vi "UHR-Fleezers Control (host) - 12.4.vi"() -> ()   [LabVIEW 2012] (continued)
        n1557 = Divide(x=w2246, y=w2245) -> (x/y=w2244:dbl)
        n1558 = Multiply(x=i16 10, y=w2223) -> (x*y=w2221:i16)
        n1559 = Multiply(x="N APD Samp/step", y=w2244) -> (x*y=w2243:dbl)
        "Cycles/step (MCL)" <- w2243
        n1560 = Divide(x=w2221, y=w2220) -> (x/y=→"Actual MCL Inc (V)":dbl)
        n1561 = Multiply(x="N APD Samp/step", y="Scan steps (MCL)") -> (x*y=w2235:dbl)
        n1562 = local read "APD Samples/FIFO Acq."() -> (w2232:dbl)
        n1563 = Multiply(x=w2235, y=u64 2) -> (x*y=w2234:dbl)
        "Data points/scan (f+b)" <- w2234
        n1564 = Multiply(x=w2234, y=w2225) -> (x*y=w2252:dbl)
        "Data points/scans (MCL)" <- w2252
        n1565 = Multiply(x=w2233, y=w2234) -> (x*y=w2226:dbl)
        "Time/f+b scan (s) (MCL)" <- w2226
        n1566 = Divide(x=w2252, y=w2232) -> (x/y=→"N sets should be saved (MCL)":dbl)
        n1567 = Multiply(x=w2226, y=w2225) -> (x*y=→"Total Time (s)":dbl)
        n1568 = Not(x="Fast Scan Dir") -> (.not. x?=w2230:bool)
        n1569 = xnode "Read/Write Control"("FPGA VI Reference In"=w2256, "error in"=w2255, "Scan steps (MCL)"="Scan steps (MCL)", "Number of scans (MCL)"=w2225, "Cycles per step (MCL)"=w2243, "Scan freq.  increment (MCL)"=w2223, "1D or 2D Scan?"="2D or 1D Scan", "MCL Scan Axis"=w2230, "Cont. Scan (MCL)"="Continuous MCL Scanning") -> ("error out"=w2254:errorcluster)  [unwired: 1 out]
      }
      event "Read Cal": Value Change {
        w2258 = 1000.0 ("y")
        n1570 = event-data() -> ()  [unwired: 7 out]
        n1571 = local read "Save file name"() -> (w2283:path)
        n1572 = local write "Read Cal"(FALSE ("Read Cal")) -> ()
        n1573 = Strip Path(path=w2283) -> (stripped path=w2282:path)  [unwired: 1 out]
        n1574 = Path To String(path=w2282) -> (string=w2281:string)
        n1575 = Concatenate Strings(w2281, "\\current.cal" ("string")) -> (w2279:string)
        n1576 = String To Path(string=w2279) -> (path=w2278:path)
        n1577 = Open/Create/Replace File(file path (use dialog)=w2278, operation (0:open)=T27."open", access (0:read/write)=enum16{"read/write", "read-only", "write-only"}."read-only") -> (refnum out=w2286:refnum<file>, error out=w2272:errorcluster)  [unwired: 1 in, 3 out]
        n1578 = Deny Access(4:w2272, 7:w2286) -> (0:w2271:errorcluster, 3:w2277:refnum<file>)  [unwired: 1 out]
        n1579 = Read from Binary File(5:0.0, 8:w2271, 9:T26."big-endian, network order" ("byte order (0:big-endian, network order)"), 10:-1 ("count (1)"), 11:w2277) -> (0:w2270:errorcluster, 2:w2268:dbl[], 3:w2273:refnum<file>)  [unwired: 2 out]
        n1580 = Array To Cluster(array=w2268) -> (cluster=w2267:T29)
        n1581 = Unbundle(w2267) -> ("[0]"=w2266:dbl, "[1]"=w2265:dbl, "[2]"=w2264:dbl, "[3]"=w2263:dbl, "[4]"=w2262:dbl, "[5]"=w2261:dbl)
        n1582 = Close File(refnum=w2273, error in=w2270) -> (error out=→"Read cal error":errorcluster)  [unwired: 1 out]
        n1583 = Multiply(x=w2261, y=w2258) -> (x*y=w2259:dbl)
        n1584 = local write "T2 kappa_x (pN/nm)"(w2263) -> ()
        n1585 = local write "T1 kappa_x (pN/nm)"(w2264) -> ()
        n1586 = local write "T1 alpha_x (nm/V)"(w2266) -> ()
        n1587 = local write "T2 alpha_x (nm/V)"(w2265) -> ()
        n1588 = Multiply(x=w2262, y=w2258) -> (x*y=w2260:dbl)
        n1589 = local write "T1 offset_x (mV)"(w2260) -> ()
        n1590 = local write "T2 offset_x (mV)"(w2259) -> ()
      }
      event "Abort MCL Scan": Value Change {
        n1591 = event-data() -> ()  [unwired: 7 out]
        n1592 = local write "MCL Scanning"(FALSE ("MCL Scanning")) -> ()
        n1593 = xnode "Read/Write Control"("FPGA VI Reference In"=w2291, "error in"=w2290, "Abort scan (MCL)"="Abort MCL Scan") -> ("error out"=w2289:errorcluster)  [unwired: 1 out]
      }
      event "Update Count (MCL)": Value Change {
        n1594 = event-data() -> ()  [unwired: 7 out]
        n1595 = xnode "Read/Write Control"("FPGA VI Reference In"=w2295, "error in"=w2294, "MCL count"="Update Count (MCL)") -> ("error out"=w2293:errorcluster)  [unwired: 1 out]
      }
      event "+ phase (MCL)", "- phase (MCL)": Value Change {
        n1596 = event-data() -> ()  [unwired: 7 out]
        n1597 = Or(x="- phase (MCL)", y="+ phase (MCL)") -> (x .or. y?=w2298:bool)
        n1598 = Negate(x="Phase adjust (MCL)") -> (-x=w2304:i16)
        n1599 = Select(t=w2304, s="+ phase (MCL)", f="Phase adjust (MCL)") -> (s? t:f=w2302:i16)
        n1600 = xnode "Read/Write Control"("FPGA VI Reference In"=w2306, "error in"=w2305, "Phase count adjustment (MCL)"=w2302) -> ("FPGA VI Reference Out"=w2299:T19, "error out"=w2300:errorcluster)
        n1601 = xnode "Read/Write Control"("FPGA VI Reference In"=w2299, "error in"=w2300, "+ phase (MCL)"=w2298) -> ("error out"=w2297:errorcluster)  [unwired: 1 out]
      }
      event "Abort AOD Scan": Value Change {
        n1602 = event-data() -> ()  [unwired: 7 out]
        n1603 = xnode "Read/Write Control"("FPGA VI Reference In"=w2310, "error in"=w2309, "Abort scan"="Abort AOD Scan") -> ("error out"=w2308:errorcluster)  [unwired: 1 out]
      }
      event "Continuous AOD Scanning": Value Change {
        n1604 = event-data() -> ()  [unwired: 7 out]
        n1605 = xnode "Read/Write Control"("FPGA VI Reference In"=w2314, "error in"=w2313, "Cont. Scan"="Continuous AOD Scanning") -> ("error out"=w2312:errorcluster)  [unwired: 1 out]
      }
      event "Index": Value Change {
        n1606 = event-data() -> ()  [unwired: 7 out]
        n1607 = call "Create new save file.vi"("Insert"="", "Ext"=".dat" ("string"), "Index In"="Index") -> ("Path Out"=→"Save file name":path, "Index Out"=w2315:dbl)
        "Save index" <- w2315
        n1608 = local write "Index"(w2315) -> ()
      }
      event "AO1", "AO2": Value Change {
        w2330 = 10.0 ("y")
        w2329 = 32767.0 ("y")
        n1609 = event-data() -> ()  [unwired: 7 out]
        n1610 = local read "AO2"() -> (w2328:dbl)
        n1611 = local read "AO1"() -> (w2325:dbl)
        n1612 = Multiply(x=w2325, y=w2329) -> (x*y=w2324:dbl)
        n1613 = Multiply(x=w2328, y=w2329) -> (x*y=w2327:dbl)
        n1614 = Divide(x=w2324, y=w2330) -> (x/y=w2323:dbl)
        n1615 = Divide(x=w2327, y=w2330) -> (x/y=w2326:dbl)
        n1616 = To Word Integer(number=w2323) -> (16bit integer=w2331:i16)
        n1617 = To Word Integer(number=w2326) -> (16bit integer=w2332:i16)
        n1618 = xnode "Read/Write Control"("FPGA VI Reference In"=w2322, "error in"=w2321, "AO1"=w2331, "AO2"=w2332) -> ("error out"=w2320:errorcluster)  [unwired: 1 out]
      }
      event "Inject Pump 1": Value Change {
        n1619 = event-data() -> ()  [unwired: 7 out]
        n1620 = local read "Use Harvard pumps\nfor beads (else Chemyx)"() -> (w2334:bool)
        n1621 = case shown="True" w2334 {
          tunnel: "Inject Pump 1" -> [w2338 w2376]
          tunnel: w2333 -> [_ w2377]
          frame False {
            n1622 = local read "Pump write delay (ms)"() -> (w2337:dbl)
            n1623 = local read "Chemyx Syringe Pump Serial Port"() -> (w2336:refnum<visa-resource-name>)
            n1624 = case shown="True" w2338 {
              tunnel: w2337 -> [w2344 w2358]
              tunnel: w2336 -> [w2341 w2357]
              frame False {
                n1625 = flat-sequence {
                  tunnel: w2341 -> [w2345]
                  tunnel: [w2345] -> w2342
                  tunnel: w2344 -> [_]
                  tunnel: [w2348] -> w2343
                  tunnel: w2342 -> [w2348]
                  tunnel: w2343 -> [w2349]
                  tunnel: [w2349] -> w2339
                  tunnel: [w2351] -> w2340
                  tunnel: w2339 -> [w2351]
                  tunnel: w2340 -> [w2353]
                  frame #0 {
                    n1626 = call "Write to pump.vi"("string"="enter pump1", "VISA resource name"=w2345) -> ()  [unwired: 1 out]
                  }
                  frame #1 {
                    n1627 = Wait (ms)(milliseconds to wait="Pump pause delay (ms)") -> ()  [unwired: 1 out]
                  }
                  frame #2 {
                    n1628 = call "Write to pump.vi"("string"="stop", "VISA resource name"=w2349) -> ()  [unwired: 1 out]
                  }
                  frame #3 {
                    n1629 = Wait (ms)(milliseconds to wait=u32 500) -> ()  [unwired: 1 out]
                  }
                  frame #4 {
                    n1630 = call "Write to pump.vi"("string"="stop", "VISA resource name"=w2353) -> ()  [unwired: 1 out]
                  }
                }
              }
              frame True {
                n1631 = flat-sequence {
                  tunnel: w2357 -> [w2367]
                  tunnel: w2358 -> [w2362]
                  tunnel: w2358 -> [w2369]
                  tunnel: w2357 -> [w2370]
                  tunnel: [w2370] -> w2355
                  tunnel: [w2372] -> w2356
                  tunnel: w2355 -> [w2372]
                  tunnel: w2356 -> [w2374]
                  frame #0 {
                    n1632 = local read "All Pump Parameters"() -> (w2361:T5)
                    n1633 = Unbundle By Name(w2361) -> ("Pump 1"=w2368:T30)
                    n1634 = call "Set pump parameters.vi"("Pump write delay (ms)"=w2362, "Volume (uL)"="Ch 1 Inject Volume (uL)", "Rate (uL/h)"="Ch 1 Inject Rate (ul/h)", "Units"=4.0, "Pump #"=1.0, "Pump Parameters In"=w2368, "VISA resource name"=w2367) -> ("Pump Parameters Out"=w2360:T30)  [unwired: 3 in]
                    n1635 = Bundle By Name(cluster=w2361, "Pump 1"=w2360) -> (w2359:T5)
                    n1636 = local write "All Pump Parameters"(w2359) -> ()
                  }
                  frame #1 {
                    n1637 = Wait (ms)(milliseconds to wait=w2369) -> ()  [unwired: 1 out]
                  }
                  frame #2 {
                    n1638 = call "Write to pump.vi"("string"="start", "VISA resource name"=w2370) -> ()  [unwired: 1 out]
                  }
                  frame #3 {
                    n1639 = Wait (ms)(milliseconds to wait=u32 500) -> ()  [unwired: 1 out]
                  }
                  frame #4 {
                    n1640 = call "Write to pump.vi"("string"="start", "VISA resource name"=w2374) -> ()  [unwired: 1 out]
                  }
                }
              }
            }
          }
          frame True {
            n1641 = case shown="False" w2376 {
              tunnel: w2377 -> [w2378 w2388]
              frame False {
                n1642 = flat-sequence {
                  tunnel: w2378 -> [w2380]
                  frame #0 {
                    n1643 = local write "Flushing P1"(FALSE ("Flushing P1")) -> ()
                    n1644 = Concatenate Strings("stop" ("string"), "\r") -> (w2382:string)
                    n1645 = VISA Write(VISA resource name=w2380, write buffer=w2382) -> ()  [unwired: 1 in, 3 out]
                  }
                  frame #1 {
                    n1646 = property on="Clear Volume P1" class="Bool (strict)"("Val(Sgnl)"=TRUE ("Value (Signaling)")) -> ()  [unwired: 2 in, 2 out]
                  }
                }
              }
              frame True {
                n1647 = local read "Normal Flow Rate (ul/h) P1"() -> (w2386:dbl)
                n1648 = Number To Decimal String(number=w2386) -> (decimal integer string=w2392:string)  [unwired: 1 in]
                n1649 = Concatenate Strings("irate  " ("string"), w2392, " u/h" ("string"), "\r") -> (w2390:string)
                n1650 = VISA Write(VISA resource name=w2388, write buffer=w2390) -> (VISA resource name out=w2387:refnum<visa-resource-name>)  [unwired: 1 in, 2 out]
                n1651 = Concatenate Strings("irun" ("string"), "\r") -> (w2394:string)
                n1652 = VISA Write(VISA resource name=w2387, write buffer=w2394) -> ()  [unwired: 1 in, 3 out]
              }
            }
          }
        }
      }
      event "Inject Pump 3": Value Change {
        n1653 = event-data() -> ()  [unwired: 7 out]
        n1654 = local read "Use Harvard pumps\nfor beads (else Chemyx)"() -> (w2397:bool)
        n1655 = case shown="True" w2397 {
          tunnel: "Inject Pump 3" -> [w2401 w2440]
          tunnel: w2396 -> [_ w2439]
          frame False {
            n1656 = local read "Pump write delay (ms)"() -> (w2400:dbl)
            n1657 = case shown="True" w2401 {
              tunnel: w2400 -> [w2407 w2421]
              tunnel: "Chemyx Syringe Pump Serial Port" -> [w2404 w2420]
              frame False {
                n1658 = flat-sequence {
                  tunnel: w2404 -> [w2408]
                  tunnel: [w2408] -> w2405
                  tunnel: w2407 -> [_]
                  tunnel: [w2411] -> w2406
                  tunnel: w2405 -> [w2411]
                  tunnel: w2406 -> [w2412]
                  tunnel: [w2412] -> w2402
                  tunnel: [w2414] -> w2403
                  tunnel: w2402 -> [w2414]
                  tunnel: w2403 -> [w2416]
                  frame #0 {
                    n1659 = call "Write to pump.vi"("string"="enter pump3", "VISA resource name"=w2408) -> ()  [unwired: 1 out]
                  }
                  frame #1 {
                    n1660 = local read "Pump pause delay (ms)"() -> (w2410:u32)
                    n1661 = Wait (ms)(milliseconds to wait=w2410) -> ()  [unwired: 1 out]
                  }
                  frame #2 {
                    n1662 = call "Write to pump.vi"("string"="stop", "VISA resource name"=w2412) -> ()  [unwired: 1 out]
                  }
                  frame #3 {
                    n1663 = Wait (ms)(milliseconds to wait=u32 0) -> ()  [unwired: 1 out]
                  }
                  frame #4 {
                    n1664 = call "Write to pump.vi"("string"="stop", "VISA resource name"=w2416) -> ()  [unwired: 1 out]
                  }
                }
              }
              frame True {
                n1665 = flat-sequence {
                  tunnel: w2420 -> [w2430]
                  tunnel: w2421 -> [w2425]
                  tunnel: w2421 -> [w2432]
                  tunnel: w2420 -> [w2433]
                  tunnel: [w2433] -> w2419
                  tunnel: [w2436] -> w2418
                  tunnel: w2419 -> [w2436]
                  tunnel: w2418 -> [w2437]
                  frame #0 {
                    n1666 = local read "All Pump Parameters"() -> (w2424:T5)
                    n1667 = Unbundle By Name(w2424) -> ("Pump 3"=w2431:T30)
                    n1668 = call "Set pump parameters.vi"("Pump write delay (ms)"=w2425, "Volume (uL)"="Ch 3 Inject Volume (uL)", "Rate (uL/h)"="Ch 3 Inject Rate (ul/h)", "Units"=4.0, "Pump #"=3.0, "Pump Parameters In"=w2431, "VISA resource name"=w2430) -> ("Pump Parameters Out"=w2423:T30)  [unwired: 3 in]
                    n1669 = Bundle By Name(cluster=w2424, "Pump 3"=w2423) -> (w2422:T5)
                    n1670 = local write "All Pump Parameters"(w2422) -> ()
                  }
                  frame #1 {
                    n1671 = Wait (ms)(milliseconds to wait=w2432) -> ()  [unwired: 1 out]
                  }
                  frame #2 {
                    n1672 = call "Write to pump.vi"("string"="start", "VISA resource name"=w2433) -> ()  [unwired: 1 out]
                  }
                  frame #3 {
                    n1673 = Wait (ms)(milliseconds to wait=u32 500) -> ()  [unwired: 1 out]
                  }
                  frame #4 {
                    n1674 = call "Write to pump.vi"("string"="start", "VISA resource name"=w2437) -> ()  [unwired: 1 out]
                  }
                }
              }
            }
          }
          frame True {
            n1675 = case shown="False" w2440 {
              tunnel: w2439 -> [w2441 w2448]
              frame False {
                n1676 = flat-sequence {
                  tunnel: w2441 -> [w2443]
                  frame #0 {
                    n1677 = local write "Flushing P3"(FALSE ("Flushing P3")) -> ()
                    n1678 = Concatenate Strings("stop" ("string"), "\r") -> (w2445:string)
                    n1679 = VISA Write(VISA resource name=w2443, write buffer=w2445) -> ()  [unwired: 1 in, 3 out]
                  }
                  frame #1 {
                    n1680 = property on="Clear Volume P3" class="Bool (strict)"("Val(Sgnl)"=TRUE ("Value (Signaling)")) -> ()  [unwired: 2 in, 2 out]
                  }
                }
              }
              frame True {
                n1681 = local read "Normal Flow Rate (ul/h) P3"() -> (w2449:dbl)
                n1682 = Number To Decimal String(number=w2449) -> (decimal integer string=w2455:string)  [unwired: 1 in]
                n1683 = Concatenate Strings("irate  " ("string"), w2455, " u/h" ("string"), "\r") -> (w2453:string)
                n1684 = VISA Write(VISA resource name=w2448, write buffer=w2453) -> (VISA resource name out=w2451:refnum<visa-resource-name>)  [unwired: 1 in, 2 out]
                n1685 = Concatenate Strings("irun" ("string"), "\r") -> (w2457:string)
                n1686 = VISA Write(VISA resource name=w2451, write buffer=w2457) -> ()  [unwired: 1 in, 3 out]
              }
            }
          }
        }
      }
      event "Inject Pump 2": Value Change {
        n1687 = event-data() -> ()  [unwired: 7 out]
        n1688 = local read "Pump write delay (ms)"() -> (w2461:dbl)
        n1689 = flat-sequence {
          tunnel: w2459 -> [w2474]
          tunnel: w2461 -> [w2470]
          tunnel: "Inject Pump 2" -> [_]
          tunnel: w2461 -> [w2476]
          tunnel: w2459 -> [w2477]
          frame #0 {
            n1690 = local read "All Pump Parameters"() -> (w2469:T5)
            n1691 = Multiply(x=60.0, y="Flush Center Ch Rate (ul/m)") -> (x*y=w2466:dbl)
            n1692 = Unbundle By Name(w2469) -> ("Pump 2"=w2475:T30)
            n1693 = call "Set pump parameters.vi"("Pump write delay (ms)"=w2470, "Volume (uL)"="Flush Center Ch Volume (uL)", "Rate (uL/h)"=w2466, "Units"=3.0, "Pump #"=2.0, "Pump Parameters In"=w2475, "VISA resource name"=w2474) -> ("Pump Parameters Out"=w2468:T30)  [unwired: 3 in]
            n1694 = Bundle By Name(cluster=w2469, "Pump 2"=w2468) -> (w2467:T5)
            n1695 = local write "All Pump Parameters"(w2467) -> ()
            n1696 = Add(x="Flush Center Ch Volume (uL)", y="Total Volume\nFlushed (uL)") -> (x+y=w2463:dbl)
            n1697 = local write "Total Volume\nFlushed (uL)"(w2463) -> ()
          }
          frame #1 {
            n1698 = Wait (ms)(milliseconds to wait=w2476) -> ()  [unwired: 1 out]
          }
          frame #2 {
            n1699 = call "Write to pump.vi"("string"="start", "VISA resource name"=w2477) -> ()  [unwired: 1 out]
          }
        }
        n1700 = local read "Chemyx Syringe Pump Serial Port"() -> (w2459:refnum<visa-resource-name>)
      }
      event "Sample Channel\nFlow": Value Change {
        n1701 = event-data() -> ()  [unwired: 7 out]
        n1702 = Select(t="irun" ("string"), s="Sample Channel\nFlow", f="stop" ("string")) -> (s? t:f=w2481:string)
        n1703 = Concatenate Strings(w2481, "\r") -> (w2484:string)
        n1704 = VISA Write(VISA resource name=w2479, write buffer=w2484) -> ()  [unwired: 1 in, 3 out]
      }
      event "Start Flow": Value Change {
        n1705 = event-data() -> ()  [unwired: 7 out]
        n1706 = local write "Sample Channel\nFlow"(TRUE ("Sample Channel\nFlow")) -> ()
        n1707 = local write "Start Flow"(FALSE ("Start Flow")) -> ()
        n1708 = Concatenate Strings("irun" ("string"), "\r") -> (w2490:string)
        n1709 = VISA Write(VISA resource name=w2486, write buffer=w2490) -> ()  [unwired: 1 in, 3 out]
      }
      event "Stop Flow": Value Change {
        w2492 = FALSE ("Stop Flow")
        n1710 = event-data() -> ()  [unwired: 7 out]
        n1711 = local write "Stop Flow"(w2492) -> ()
        n1712 = local write "Sample Channel\nFlow"(w2492) -> ()
        n1713 = Concatenate Strings("stop" ("string"), "\r") -> (w2495:string)
        n1714 = VISA Write(VISA resource name=w2493, write buffer=w2495) -> ()  [unwired: 1 in, 3 out]
      }
      event "Flow rate (uL/h)": Value Change {
        n1715 = event-data() -> ()  [unwired: 7 out]
        n1716 = Number To Decimal String(number="Flow rate (uL/h)") -> (decimal integer string=w2502:string)  [unwired: 1 in]
        n1717 = Concatenate Strings("irate  " ("string"), w2502, " u/h" ("string"), "\r") -> (w2501:string)
        n1718 = VISA Write(VISA resource name=w2498, write buffer=w2501) -> ()  [unwired: 1 in, 3 out]
      }
      event "Flush Sample": Value Change {
        n1719 = event-data() -> ()  [unwired: 7 out]
        n1720 = flat-sequence {
          tunnel: w2507 -> [w2535]
          tunnel: [w2515] -> w2506
          tunnel: [w2509] -> w2504
          tunnel: w2506 -> [w2539]
          tunnel: [w2539] -> w2505
          tunnel: w2504 -> [w2538]
          tunnel: w2505 -> [w2544]
          frame #0 {
            # "set paramaters (rate, volume) for flush, clear volume"
            n1721 = Number To Decimal String(number="Flush rate (uL/m)") -> (decimal integer string=w2531:string)  [unwired: 1 in]
            n1722 = Concatenate Strings("irate  " ("string"), w2531, " u/m" ("string"), "\r") -> (w2533:string)
            n1723 = VISA Write(VISA resource name=w2535, write buffer=w2533) -> (VISA resource name out=w2529:refnum<visa-resource-name>)  [unwired: 1 in, 2 out]
            n1724 = Reciprocal(x="Flush rate (uL/m)") -> (1/x=w2512:dbl)
            n1725 = Number To Decimal String(number="Volume (uL)") -> (decimal integer string=w2520:string)  [unwired: 1 in]
            n1726 = Multiply(x="Volume (uL)", y=w2512) -> (x*y=w2511:dbl)
            n1727 = Concatenate Strings("tvolume  " ("string"), w2520, " u" ("string"), "\r") -> (w2518:string)
            n1728 = Multiply(x=w2511, y=60000.0) -> (x*y=w2509:dbl)
            n1729 = VISA Write(VISA resource name=w2529, write buffer=w2518) -> (VISA resource name out=w2517:refnum<visa-resource-name>)  [unwired: 1 in, 2 out]
            n1730 = Concatenate Strings("cvolume" ("string"), "\r") -> (w2516:string)
            n1731 = VISA Write(VISA resource name=w2517, write buffer=w2516) -> (VISA resource name out=w2527:refnum<visa-resource-name>)  [unwired: 1 in, 2 out]
            n1732 = Concatenate Strings("irun" ("string"), "\r") -> (w2525:string)
            n1733 = VISA Write(VISA resource name=w2527, write buffer=w2525) -> (VISA resource name out=w2515:refnum<visa-resource-name>)  [unwired: 1 in, 2 out]
          }
          frame #1 {
            # "Have to wait until\nflow is done to reset\nrate"
            n1734 = Add(x=w2538, y=100.0) -> (x+y=w2537:dbl)
            n1735 = Wait (ms)(milliseconds to wait=w2537) -> ()  [unwired: 1 out]
          }
          frame #2 {
            # "reset flow rate to usual flow rate"
            n1736 = local read "Flow rate (uL/h)"() -> (w2550:dbl)
            n1737 = Number To Decimal String(number=w2550) -> (decimal integer string=w2548:string)  [unwired: 1 in]
            n1738 = Concatenate Strings("irate  " ("string"), w2548, " u/h" ("string"), "\r") -> (w2546:string)
            n1739 = VISA Write(VISA resource name=w2544, write buffer=w2546) -> (VISA resource name out=w2540:refnum<visa-resource-name>)  [unwired: 1 in, 2 out]
            n1740 = Concatenate Strings("cvolume" ("string"), "\r") -> (w2541:string)
            n1741 = VISA Write(VISA resource name=w2540, write buffer=w2541) -> ()  [unwired: 1 in, 3 out]
          }
        }
      }
      event "Flush Pump 3": Value Change {
        n1742 = event-data() -> ()  [unwired: 7 out]
        n1743 = flat-sequence {
          tunnel: w2551 -> [w2554]
          frame #0 {
            # "set paramaters (rate, volume) for flush, clear volume"
            n1744 = Number To Decimal String(number="Flush rate (uL/m) P3") -> (decimal integer string=w2576:string)  [unwired: 1 in]
            n1745 = local write "Inject Pump 3"(TRUE ("Inject Pump 3")) -> ()
            n1746 = Concatenate Strings("irate  " ("string"), w2576, " u/m" ("string"), "\r") -> (w2578:string)
            n1747 = VISA Write(VISA resource name=w2554, write buffer=w2578) -> (VISA resource name out=w2574:refnum<visa-resource-name>)  [unwired: 1 in, 2 out]
            n1748 = Reciprocal(x="Flush rate (uL/m) P3") -> (1/x=w2558:dbl)
            n1749 = Number To Decimal String(number="Volume (uL) P3") -> (decimal integer string=w2565:string)  [unwired: 1 in]
            n1750 = Multiply(x="Volume (uL) P3", y=w2558) -> (x*y=w2557:dbl)
            n1751 = Concatenate Strings("tvolume  " ("string"), w2565, " u" ("string"), "\r") -> (w2563:string)
            n1752 = Multiply(x=w2557, y=60.0) -> (x*y=→"HP3 Flush Time (s)":dbl)
            n1753 = VISA Write(VISA resource name=w2574, write buffer=w2563) -> (VISA resource name out=w2562:refnum<visa-resource-name>)  [unwired: 1 in, 2 out]
            n1754 = Concatenate Strings("cvolume" ("string"), "\r") -> (w2561:string)
            n1755 = VISA Write(VISA resource name=w2562, write buffer=w2561) -> (VISA resource name out=w2572:refnum<visa-resource-name>)  [unwired: 1 in, 2 out]
            n1756 = Concatenate Strings("irun" ("string"), "\r") -> (w2570:string)
            n1757 = VISA Write(VISA resource name=w2572, write buffer=w2570) -> ()  [unwired: 1 in, 3 out]
          }
          frame #1 {
            "Flushing P3" <- TRUE ("Flushing P3")
          }
        }
      }
      event "Flush Pump 1": Value Change {
        n1758 = event-data() -> ()  [unwired: 7 out]
        n1759 = flat-sequence {
          tunnel: [w2592] -> w2582
          tunnel: w2581 -> [w2585]
          tunnel: w2582 -> [_]
          frame #0 {
            # "set paramaters (rate, volume) for flush, clear volume"
            n1760 = local write "Inject Pump 1"(TRUE ("Inject Pump 1")) -> ()
            n1761 = Number To Decimal String(number="Flush rate (uL/m) P1") -> (decimal integer string=w2608:string)  [unwired: 1 in]
            n1762 = Concatenate Strings("irate  " ("string"), w2608, " u/m" ("string"), "\r") -> (w2610:string)
            n1763 = VISA Write(VISA resource name=w2585, write buffer=w2610) -> (VISA resource name out=w2606:refnum<visa-resource-name>)  [unwired: 1 in, 2 out]
            n1764 = Reciprocal(x="Flush rate (uL/m) P1") -> (1/x=w2589:dbl)
            n1765 = Number To Decimal String(number="Volume (uL) P1") -> (decimal integer string=w2597:string)  [unwired: 1 in]
            n1766 = Multiply(x="Volume (uL) P1", y=w2589) -> (x*y=w2588:dbl)
            n1767 = Concatenate Strings("tvolume  " ("string"), w2597, " u" ("string"), "\r") -> (w2595:string)
            n1768 = Multiply(x=w2588, y=60.0) -> (x*y=→"HP1 Flush Time (s)":dbl)
            n1769 = VISA Write(VISA resource name=w2606, write buffer=w2595) -> (VISA resource name out=w2594:refnum<visa-resource-name>)  [unwired: 1 in, 2 out]
            n1770 = Concatenate Strings("cvolume" ("string"), "\r") -> (w2593:string)
            n1771 = VISA Write(VISA resource name=w2594, write buffer=w2593) -> (VISA resource name out=w2604:refnum<visa-resource-name>)  [unwired: 1 in, 2 out]
            n1772 = Concatenate Strings("irun" ("string"), "\r") -> (w2602:string)
            n1773 = VISA Write(VISA resource name=w2604, write buffer=w2602) -> (VISA resource name out=w2592:refnum<visa-resource-name>)  [unwired: 1 in, 2 out]
          }
          frame #1 {
            "Flushing P1" <- TRUE ("Flushing P3")
          }
        }
      }
      event "Clear Volume": Value Change {
        n1774 = event-data() -> ()  [unwired: 7 out]
        n1775 = Concatenate Strings("cvolume" ("string"), "\r") -> (w2614:string)
        n1776 = VISA Write(VISA resource name=w2613, write buffer=w2614) -> ()  [unwired: 1 in, 3 out]
      }
      event "Clear Volume P3": Value Change {
        n1777 = event-data() -> ()  [unwired: 7 out]
        n1778 = Concatenate Strings("cvolume" ("string"), "\r") -> (w2620:string)
        n1779 = VISA Write(VISA resource name=w2619, write buffer=w2620) -> ()  [unwired: 1 in, 3 out]
        n1780 = local write "Clear Volume P3"(FALSE ("Clear Volume P3")) -> ()
      }
      event "Clear Volume P1": Value Change {
        n1781 = event-data() -> ()  [unwired: 7 out]
        n1782 = Concatenate Strings("cvolume" ("string"), "\r") -> (w2625:string)
        n1783 = local write "Clear Volume P1"(FALSE ("Clear Volume P1")) -> ()
        n1784 = VISA Write(VISA resource name=w2624, write buffer=w2625) -> ()  [unwired: 1 in, 3 out]
      }
      event "Display On P3": Value Change {
        n1785 = event-data() -> ()  [unwired: 7 out]
        n1786 = Select(t="dim 100", s="Display On P3", f="dim 0") -> (s? t:f=w2631:string)
        n1787 = Concatenate Strings(w2631, "\r") -> (w2633:string)
        n1788 = VISA Write(VISA resource name=w2628, write buffer=w2633) -> ()  [unwired: 1 in, 3 out]
      }
      event "Display On P1": Value Change {
        n1789 = event-data() -> ()  [unwired: 7 out]
        n1790 = Select(t="dim 100", s="Display On P1", f="dim 0") -> (s? t:f=w2638:string)
        n1791 = Concatenate Strings(w2638, "\r") -> (w2640:string)
        n1792 = VISA Write(VISA resource name=w2635, write buffer=w2640) -> ()  [unwired: 1 in, 3 out]
      }
      event "Retract Pump 3": Value Change {
        n1793 = event-data() -> ()  [unwired: 7 out]
        n1794 = local write "Retract Pump 3"(FALSE ("Retract Pump 3")) -> ()
        n1795 = case shown="True" "Retract Pump 3" {
          tunnel: w2642 -> [_ w2645]
          frame False {
          }
          frame True {
            n1796 = Number To Decimal String(number="Retract Rate (uL/m)") -> (decimal integer string=w2663:string)  [unwired: 1 in]
            n1797 = Concatenate Strings("wrate  " ("string"), w2663, " u/m" ("string"), "\r") -> (w2665:string)
            n1798 = VISA Write(VISA resource name=w2645, write buffer=w2665) -> (VISA resource name out=w2656:refnum<visa-resource-name>)  [unwired: 1 in, 2 out]
            n1799 = Number To Decimal String(number="Retract Vol 3 (uL)") -> (decimal integer string=w2658:string)  [unwired: 1 in]
            n1800 = Concatenate Strings("tvolume  " ("string"), w2658, " u" ("string"), "\r") -> (w2655:string)
            n1801 = VISA Write(VISA resource name=w2656, write buffer=w2655) -> (VISA resource name out=w2651:refnum<visa-resource-name>)  [unwired: 1 in, 2 out]
            n1802 = Concatenate Strings("cvolume" ("string"), "\r") -> (w2652:string)
            n1803 = VISA Write(VISA resource name=w2651, write buffer=w2652) -> (VISA resource name out=w2646:refnum<visa-resource-name>)  [unwired: 1 in, 2 out]
            n1804 = Concatenate Strings("wrun" ("string"), "\r") -> (w2647:string)
            n1805 = VISA Write(VISA resource name=w2646, write buffer=w2647) -> ()  [unwired: 1 in, 3 out]
          }
        }
      }
      event "Retract Pump 1": Value Change {
        n1806 = event-data() -> ()  [unwired: 7 out]
        n1807 = local write "Retract Pump 1"(FALSE ("Retract Pump 1")) -> ()
        n1808 = case shown="True" "Retract Pump 1" {
          tunnel: w2667 -> [_ w2672]
          frame False {
          }
          frame True {
            n1809 = local read "Retract Rate (uL/m)"() -> (w2670:dbl)
            n1810 = Number To Decimal String(number=w2670) -> (decimal integer string=w2688:string)  [unwired: 1 in]
            n1811 = Concatenate Strings("wrate  " ("string"), w2688, " u/m" ("string"), "\r") -> (w2690:string)
            n1812 = VISA Write(VISA resource name=w2672, write buffer=w2690) -> (VISA resource name out=w2682:refnum<visa-resource-name>)  [unwired: 1 in, 2 out]
            n1813 = Number To Decimal String(number="Retract Vol 1 (uL)") -> (decimal integer string=w2684:string)  [unwired: 1 in]
            n1814 = Concatenate Strings("tvolume  " ("string"), w2684, " u" ("string"), "\r") -> (w2681:string)
            n1815 = VISA Write(VISA resource name=w2682, write buffer=w2681) -> (VISA resource name out=w2678:refnum<visa-resource-name>)  [unwired: 1 in, 2 out]
            n1816 = Concatenate Strings("cvolume" ("string"), "\r") -> (w2679:string)
            n1817 = VISA Write(VISA resource name=w2678, write buffer=w2679) -> (VISA resource name out=w2673:refnum<visa-resource-name>)  [unwired: 1 in, 2 out]
            n1818 = Concatenate Strings("wrun" ("string"), "\r") -> (w2674:string)
            n1819 = VISA Write(VISA resource name=w2673, write buffer=w2674) -> ()  [unwired: 1 in, 3 out]
          }
        }
      }
      event "Flip Green Filter": Value Change {
        n1820 = event-data() -> ()  [unwired: 7 out]
        n1821 = Not(x="Flip Green Filter") -> (.not. x?=w2692:bool)
        n1822 = local write "Flip Green Filter"(w2692) -> ()
        n1823 = flat-sequence {
          tunnel: w2700 -> [w2705]
          tunnel: w2699 -> [w2704]
          tunnel: [w2702] -> w2697
          tunnel: [w2701] -> w2696
          tunnel: [w2707] -> w2695
          tunnel: w2697 -> [w2707]
          tunnel: [w2706] -> w2694
          tunnel: w2696 -> [w2706]
          tunnel: w2695 -> [w2711]
          tunnel: w2694 -> [w2710]
          tunnel: [w2709] -> w2698
          frame #0 {
            n1824 = xnode "Read/Write Control"("FPGA VI Reference In"=w2705, "error in"=w2704, "Green Filter Flipper"=TRUE) -> ("FPGA VI Reference Out"=w2702:T19, "error out"=w2701:errorcluster)
          }
          frame #1 {
            n1825 = Wait (ms)(milliseconds to wait=u32 100) -> ()  [unwired: 1 out]
          }
          frame #2 {
            n1826 = xnode "Read/Write Control"("FPGA VI Reference In"=w2711, "error in"=w2710, "Green Filter Flipper"=FALSE) -> ("error out"=w2709:errorcluster)  [unwired: 1 out]
          }
        }
      }
      event "Pump 1 contents", "Pump 3 contents": Value Change {
        n1827 = event-data() -> ()  [unwired: 7 out]
        n1828 = local read "Pump 1 contents"() -> (→"Pump 1 cont disp":string)
        n1829 = local read "Pump 3 contents"() -> (→"Pump 3 cont disp":string)
      }
      event "Reset Trap Pos. FB": Value Change {
        n1830 = event-data() -> ()  [unwired: 7 out]
        n1831 = xnode "Read/Write Control"("FPGA VI Reference In"=w2717, "error in"=w2716, "Trap Pos. FB Reset"="Reset Trap Pos. FB") -> ()  [unwired: 2 out]
      }
      event "Rem fb disp offset": Value Change {
        n1832 = event-data() -> ()  [unwired: 7 out]
        n1833 = local write "Rem fb disp offset"(FALSE ("Rem fb disp offset")) -> ()
        n1834 = local read "Mean T1 Position (nm)"() -> (w2719:dbl)
        n1835 = local read "FB Trap Pos Offset"() -> (w2720:dbl)
        n1836 = Subtract(x=w2720, y=w2719) -> (x-y=w2718:dbl)
        n1837 = local write "FB Trap Pos Offset"(w2718) -> ()
      }
      event "Threshold (nm)": Value Change {
        n1838 = event-data() -> ()  [unwired: 7 out]
        n1839 = flat-sequence {
          tunnel: w2724 -> [w2732]
          tunnel: w2723 -> [w2731]
          tunnel: [w2725] -> w2722
          tunnel: w2722 -> [w2738]
          frame #0 {
            n1840 = xnode "Read/Write Control"("FPGA VI Reference In"=w2732, "error in"=w2731) -> ("FPGA VI Reference Out"=w2728:T19, "error out"=w2727:errorcluster, "FPGA TTrig Thresh"=w2729:i64)
            n1841 = local read "Threshold stored (nm)"() -> (w2737:dbl)
            n1842 = local read "Threshold (nm)"() -> (w2725:dbl)
            n1843 = local read "AOM X Cal (nm/MHz)"() -> (w2735:dbl)
            n1844 = Subtract(x=w2725, y=w2737) -> (x-y=w2736:dbl)
            n1845 = Divide(x=w2736, y=w2735) -> (x/y=w2733:dbl)
            n1846 = call "IR AOM freq to word.vi"("Frequency In (MHz)"=w2733) -> ("Frequency Word Out (double)"=w2734:dbl)
            n1847 = To Quad Integer(1:w2734) -> (0:w2730:i64)
            n1848 = Add(x=w2729, y=w2730) -> (x+y=w2726:i64)
            n1849 = xnode "Read/Write Control"("FPGA VI Reference In"=w2728, "error in"=w2727, "FPGA TTrig Thresh"=w2726) -> ()  [unwired: 2 out]
          }
          frame #1 {
            "Threshold stored (nm)" <- w2738
          }
        }
      }
      event "FB Trig Integrate": Value Change {
        n1850 = event-data() -> ()  [unwired: 7 out]
        n1851 = local read "FB Trig Integrate"() -> (w2740:u32)
        n1852 = xnode "Read/Write Control"("FPGA VI Reference In"=w2742, "error in"=w2741, "FB Trig Integrate"=w2740) -> ("error out"=w2739:errorcluster)  [unwired: 1 out]
      }
      event "11": Value Change {
        n1853 = event-data() -> ()  [unwired: 7 out]
        n1854 = local read "11"() -> (w2743:bool)
        n1855 = case shown="True" w2743 {
          frame False {
          }
          frame True {
            n1856 = local read "Messages"() -> (w2745:string)
            n1857 = call "Update messages.vi"("Message to add"="You kicked it up to 11!", "Old message string"=w2745) -> ("New message string"=w2746:string)
            n1858 = call <vilib>:"Beep.vi"() -> ()  [unwired: 12 in]
            n1859 = local write "Messages"(w2746) -> ()
          }
        }
      }
      event "Trap Pos. FB ON": Value Change {
        n1860 = event-data() -> ()  [unwired: 7 out]
        n1861 = xnode "Read/Write Control"("FPGA VI Reference In"=w2749, "error in"=w2748, "Force feedback"="Trap Pos. FB ON") -> ()  [unwired: 2 out]
      }
      event "Remove Action Offset": Value Change {
        n1862 = event-data() -> ()  [unwired: 7 out]
        n1863 = local write "Remove Action Offset"(FALSE ("Remove Action Offset")) -> ()
        n1864 = local read "Trap Pos. FB Mult Factor"() -> (w2754:i64)
        n1865 = local read "Trap Pos FB Action"() -> (w2752:i64)
        n1866 = local read "Trap Pos. FB Offset Factor"() -> (w2750:i64)
        n1867 = Multiply(x=w2754, y=w2752) -> (x*y=w2753:i64)
        n1868 = Add(x=w2753, y=w2750) -> (x+y=w2751:i64)
        n1869 = local write "Trap Pos. FB Offset Factor"(w2751) -> ()
        n1870 = xnode "Read/Write Control"("FPGA VI Reference In"=w2757, "error in"=w2756, "Trap Pos. FB Offset Factor"=w2751) -> ()  [unwired: 2 out]
      }
      event "Remove Unwinding Offset": Value Change {
        n1871 = event-data() -> ()  [unwired: 7 out]
        n1872 = local write "Remove Unwinding Offset"(FALSE ("Remove Action Offset")) -> ()
        n1873 = local read "Trap Pos. FB Mult Factor"() -> (w2769:i64)
        n1874 = local read "Trap Pos FB Action"() -> (w2767:i64)
        n1875 = local read "Trap Pos. FB Offset Factor"() -> (w2766:i64)
        n1876 = Multiply(x=w2769, y=w2767) -> (x*y=w2768:i64)
        n1877 = local read "Trap Pos. FB Mult Factor"() -> (w2765:i64)
        n1878 = Add(x=w2768, y=w2766) -> (x+y=w2759:i64)
        n1879 = Multiply(x=32768, y="factor") -> (x*y=w2762:dbl)
        n1880 = Multiply(x=w2762, y=w2765) -> (x*y=w2764:dbl)
        n1881 = Subtract(x=w2759, y=w2764) -> (x-y=w2763:dbl)
        n1882 = To Quad Integer(1:w2763) -> (0:w2758:i64)
        n1883 = xnode "Read/Write Control"("FPGA VI Reference In"=w2772, "error in"=w2771, "Trap Pos. FB Offset Factor"=w2758) -> ()  [unwired: 2 out]
        n1884 = local write "Trap Pos. FB Offset Factor"(w2758) -> ()
      }
      event "Trap Pos. FB Range", "Trap Pos. FB Gains", "Trap Pos. FB Mult Factor", "Trap Pos. FB Offset Factor", "Trap Pos FB Negate Action", "Trap Pos FB Monitor\nT1 or T2", "Differential FB?", "Negate Diff?": Value Change {
        n1885 = event-data() -> ()  [unwired: 7 out]
        n1886 = Unbundle By Name("Trap Pos. FB Gains") -> ("proportional gain (Kc)"=w2775:fxp<+/-,16,8>, "integral gain (Kc*Ts/Ti)"=w2774:fxp<+/-,16,8>, "derivative gain (Kc*Td/Ts)"=w2773:fxp<+/-,16,8>)
        n1887 = local read "Negate Diff?"() -> (w2780:bool)
        n1888 = Unbundle By Name("Trap Pos. FB Range") -> ("output high"=w2778:fxp<+/-,16,1>, "output low"=w2777:fxp<+/-,16,1>)
        n1889 = xnode "Read/Write Control"("FPGA VI Reference In"=w2788, "error in"=w2787, "FB2 output high"=w2778, "FB2 output low"=w2777, "P2"=w2775, "I2"=w2774, "D2"=w2773, "Trap Pos. FB Mult Factor"="Trap Pos. FB Mult Factor", "Trap Pos. FB Offset Factor"="Trap Pos. FB Offset Factor", "Trap Pos FB Negate Action"="Trap Pos FB Negate Action", "Trap Pos FB Monitor T1 or T2"="Trap Pos FB Monitor\nT1 or T2", "AI1 X Scale"="Trap Pos. AI1 X Pre-scale", "Negate Diff?"=w2780, "Diff FB Measurement?"="Differential FB?") -> ()  [unwired: 2 out]
      }
      event "Trap Pos FB SP", "Trap Pos FB SP 2", "Use SP 2": Value Change {
        n1890 = event-data() -> ()  [unwired: 7 out]
        n1891 = Select(t="Trap Pos FB SP 2", s="Use SP 2", f="Trap Pos FB SP") -> (s? t:f=w2789:fxp<+/-,16,1>)
        n1892 = xnode "Read/Write Control"("FPGA VI Reference In"=w2794, "error in"=w2793, "Trap Pos. FB SP"=w2789) -> ()  [unwired: 2 out]
      }
      event "Offset SP2 from SP1": Value Change {
        n1893 = event-data() -> ()  [unwired: 7 out]
        n1894 = local read "Trap Pos FB SP"() -> (w2797:fxp<+/-,16,1>)
        n1895 = Add(x=w2797, y="SP2 Offset") -> (x+y=w2795:fxp<+/-,16,1>)
        n1896 = property on="Trap Pos FB SP 2" class="DigNum (strict)"("Val(Sgnl)"=w2795) -> ()  [unwired: 2 in, 2 out]
        n1897 = local write "Offset SP2 from SP1"(FALSE ("Offset SP2 from SP1")) -> ()
      }
      event "Set Reading to\nSetpoint": Value Change {
        # "This is the actual PID input signal"
        n1898 = event-data() -> ()  [unwired: 7 out]
        n1899 = local write "Set Reading to\nSetpoint"(FALSE ("Set SP to Reading")) -> ()
        n1900 = xnode "Read/Write Control"("FPGA VI Reference In"=w2803, "error in"=w2802) -> ("FPGA VI Reference Out"=w2801:T19, "error out"=w2800:errorcluster, "Trap Pos FB Int-Norm Signal"=w2799:fxp<+/-,16,1>)
        n1901 = local read "Differential FB?"() -> (w2804:bool)
        n1902 = case shown="False" w2804 {
          tunnel: [w2809 w2816] -> w2806
          tunnel: w2799 -> [w2807 w2816]
          frame False {
            n1903 = local read "Trap Pos FB Monitor\nT1 or T2"() -> (w2812:bool)
            n1904 = local read "Trap X AI1 (DMA)"() -> (w2815:T13)
            n1905 = Unbundle By Name(w2815) -> ("Set 1"=w2814:fxp<+/-,16,1>, "Set 2"=w2813:fxp<+/-,16,1>)
            n1906 = Select(t=w2814, s=w2812, f=w2813) -> (s? t:f=w2811:fxp<+/-,16,1>)
            n1907 = Not(x="Set SP Using...") -> (.not. x?=w2808:bool)
            n1908 = Select(t=w2807, s=w2808, f=w2811) -> (s? t:f=w2809:fxp<+/-,16,1>)
          }
          frame True {
          }
        }
        n1909 = xnode "Read/Write Control"("FPGA VI Reference In"=w2801, "error in"=w2800, "Trap Pos. FB SP"=w2806) -> ()  [unwired: 2 out]
        n1910 = local write "Trap Pos FB SP"(w2806) -> ()
      }
      event "Trap Pos. FB Out Scale 2^n": Value Change {
        n1911 = event-data() -> ()  [unwired: 7 out]
        n1912 = Scale By Power Of 2(n="Trap Pos. FB Out Scale 2^n", x=ext 1.0) -> (x*2^n=w2817:ext)
        n1913 = property on="Trap Pos. FB Mult Factor" class="DigNum (strict)"("Val(Sgnl)"=w2817) -> ()  [unwired: 2 in, 2 out]
      }
      event "Trap Pos FB Int Count": Value Change {
        n1914 = event-data() -> ()  [unwired: 7 out]
        n1915 = xnode "Read/Write Control"("FPGA VI Reference In"=w2822, "error in"=w2821, "Trap Pos FB Int Count"="Trap Pos FB Int Count") -> ()  [unwired: 2 out]
      }
      event "Trap pos": Value Change {
        n1916 = event-data() -> ()  [unwired: 7 out]
        n1917 = case shown="True" "Trap pos" {
          frame False {
            n1918 = property on="Trap Delta Graph" class="WFGraph (strict)"("Visible"=TRUE) -> ()  [unwired: 2 in, 2 out]
            n1919 = property on="Saved trap pos" class="WFGraph (strict)"("Visible"=FALSE) -> ()  [unwired: 2 in, 2 out]
          }
          frame True {
            n1920 = property on="Saved trap pos" class="WFGraph (strict)"("Visible"=TRUE) -> ()  [unwired: 2 in, 2 out]
            n1921 = property on="Trap Delta Graph" class="WFGraph (strict)"("Visible"=FALSE) -> ()  [unwired: 2 in, 2 out]
          }
        }
      }
    }
    "error out 2" <- w1632
    n1922 = node-c288() -> ()  [unwired: 2 out]
  }
  n1923 = while "Duncan's play event loop" {
    stop <- w2829 stop-if-true
    n1924 = Create User Event(user event datatype=TRUE ("Boolean")) -> (user event=w2830:refnum<user-event>)  [unwired: 1 in, 1 out]
    n1925 = Create User Event(user event datatype=TRUE ("Boolean")) -> (user event=w2837:refnum<user-event>)  [unwired: 1 in, 1 out]
    n1926 = global write "Global for fluorescence simulation mean (30 samples), (power series).vi" "Red Signal"(w2830) -> ()
    n1927 = global write "Global for fluorescence simulation mean (30 samples), (power series).vi" "Green Signal"(w2837) -> ()
    n1928 = register-events(w2837, w2830) -> (reference out=w2836:refnum<event-registration>)  [unwired: 2 in, 1 out]
    n1929 = event shown="[1] \"Get Fluorophore\": Value Change" {
      selector: w2836 -> [_ _ _ _]
      dyn-events: _ -> [_ _ _ _]
      timeout: 100 -> [_ _ _ _]
      event Timeout {
        n1930 = event-data() -> ()  [unwired: 1 in, 2 out]
      }
      event "Get Fluorophore": Value Change {
        n1931 = event-data() -> ("OldVal"=w2839:bool)  [unwired: 1 in, 4 out]
        n1932 = case shown="True" w2839 {
          selector: w2839 -> [_ w2840]
          frame False {
          }
          frame True {
            n1933 = property on="Move to Position 3" class="Bool"("Val(Sgnl)"=w2840) -> ()  [unwired: 2 in, 2 out]
            n1934 = case shown="1" "Numeric" {
              frame 0, Default {
              }
              frame 1 {
                n1935 = property on="Green Laser ON" class="Bool (strict)"("Val(Sgnl)"=TRUE ("Value (Signaling)")) -> ()  [unwired: 2 in, 2 out]
              }
              frame 2 {
                n1936 = property on="Red Laser ON" class="Bool (strict)"("Val(Sgnl)"=TRUE) -> ()  [unwired: 2 in, 2 out]
              }
            }
          }
        }
      }
      event User Event {
        n1937 = event-data() -> ("Boolean"=w2844:bool)  [unwired: 1 in, 3 out]
        "Green Fluorophore" <- w2844
        n1938 = property on="Get Fluorophore" class="Bool (strict)"("Val(Sgnl)"=w2844) -> ()  [unwired: 2 in, 2 out]
      }
      event User Event {
        n1939 = event-data() -> ("Boolean"=w2845:bool)  [unwired: 1 in, 3 out]
        "Red Fluorophore" <- w2845
        n1940 = property on="Get Fluorophore" class="Bool (strict)"("Val(Sgnl)"=w2845) -> ()  [unwired: 2 in, 2 out]
      }
    }
    n1941 = property on="Get Fluorophore" class="Bool (strict)"("Val(Sgnl)"="Get Fluorophore") -> ()  [unwired: 2 in, 2 out]
    n1942 = Wait (ms)(milliseconds to wait=u32 100) -> ()  [unwired: 1 out]
    n1943 = local read "Stop All"() -> (w2828:bool)
    n1944 = Or(x=w2828, y="stop") -> (x .or. y?=w2829:bool)
  }
  n1945 = timed-loop "Mouse control: trap position (AOM deflection), set confocal spot from image" {
    tunnel: [w2847] -> w207
    tunnel: w13 -> [w2846]
    timing: w129 -> [_]
    timing-out: [_] -> w128
    stop <- w2847 stop-if-true
    n1946 = node-c288() -> ()  [unwired: 2 out]
    n1947 = event shown="[0] \"Pane\": Mouse Down" {
      selector: _ -> [_ _]
      dyn-events: _ -> [_ _]
      timeout: _ -> [_ _]
      tunnel: w2846 -> [w2850 _]
      event Mouse Down {
        n1948 = event-data() -> ("Time"=w2852:u32, "Coords"=w2851:T7, "Button"=w2853:u16)  [unwired: 6 out]
        n1949 = case shown="1" w2853 {
          tunnel: w2852 -> [_ _ w2959]
          tunnel: w2851 -> [_ w2890 w2957]
          tunnel: w2850 -> [_ _ w2955]
          frame 0, Default {
          }
          frame 1 {
            n1950 = property on="APD 2" class="ImageControl"() -> ("Displayed Image Position"=w2860:cluster{"Left":i32, "Top":i32})  [unwired: 2 in, 2 out]
            n1951 = property on="APD 1" class="ImageControl"() -> ("Displayed Image Position"=w2889:cluster{"Left":i32, "Top":i32})  [unwired: 2 in, 2 out]
            n1952 = property on="Detection Laser X" class="ImageControl"() -> ("Displayed Image Position"=w2886:cluster{"Left":i32, "Top":i32})  [unwired: 2 in, 2 out]
            n1953 = property on="Detection Laser Y" class="ImageControl"() -> ("Displayed Image Position"=w2885:cluster{"Left":i32, "Top":i32})  [unwired: 2 in, 2 out]
            n1954 = property on="APD 2" class="ImageControl"() -> ("Displayed Image Size"=w2859:cluster{"Width":u32, "Height":u32})  [unwired: 2 in, 2 out]
            n1955 = property on="APD 1" class="ImageControl"() -> ("Displayed Image Size"=w2887:cluster{"Width":u32, "Height":u32})  [unwired: 2 in, 2 out]
            n1956 = property on="Detection Laser X" class="ImageControl"() -> ("Displayed Image Size"=w2888:cluster{"Width":u32, "Height":u32})  [unwired: 2 in, 2 out]
            n1957 = property on="Detection Laser Y" class="ImageControl"() -> ("Displayed Image Size"=w2884:cluster{"Width":u32, "Height":u32})  [unwired: 2 in, 2 out]
            n1958 = Unbundle By Name(w2859) -> ("Width"=w2856:u32, "Height"=w2855:u32)
            n1959 = Unbundle By Name(w2860) -> ("Left"=w2858:i32, "Top"=w2857:i32)
            n1960 = Unbundle By Name(w2887) -> ("Width"=w2881:u32, "Height"=w2880:u32)
            n1961 = Unbundle By Name(w2888) -> ("Width"=w2877:u32, "Height"=w2876:u32)
            n1962 = Unbundle By Name(w2884) -> ("Width"=w2873:u32, "Height"=w2872:u32)
            n1963 = Unbundle By Name(w2889) -> ("Left"=w2883:i32, "Top"=w2882:i32)
            n1964 = Unbundle By Name(w2886) -> ("Left"=w2879:i32, "Top"=w2878:i32)
            n1965 = Unbundle By Name(w2885) -> ("Left"=w2875:i32, "Top"=w2874:i32)
            n1966 = Bundle("Left"=w2858, "Top"=w2857, "Width"=w2856, "Height"=w2855) -> (w2854:T31)  [unwired: 1 in]
            n1967 = Bundle("Left"=w2883, "Top"=w2882, "Width"=w2881, "Height"=w2880) -> (w2871:T31)  [unwired: 1 in]
            n1968 = Bundle("Left"=w2879, "Top"=w2878, "Width"=w2877, "Height"=w2876) -> (w2870:T31)  [unwired: 1 in]
            n1969 = Bundle("Left"=w2875, "Top"=w2874, "Width"=w2873, "Height"=w2872) -> (w2869:T31)  [unwired: 1 in]
            n1970 = Build Cluster Array(w2854, w2871, w2870, w2869) -> (w2868:T32)
            n1971 = for {
              tunnel: w2890 -> [w2901]
              tunnel: w2868 -> [w2902] mode=indexing
              shift-right: [w2899] -> w2866
              shift-left: TRUE -> [w2900]
              shift-right: [w2898] -> w2864
              shift-left: _ -> [w2894]
              shift-right: [w2897] -> w2863
              shift-left: _ -> [w2893]
              shift-right: [w2896] -> w2862
              shift-left: _ -> [w2892]
              shift-right: [w2895] -> w2861
              shift-left: _ -> [w2891]
              n1972 = case shown="True" w2900 {
                selector: w2900 -> [w2907 _]
                tunnel: w2902 -> [_ w2916]
                tunnel: w2901 -> [_ w2914]
                tunnel: [w2907 w2912] -> w2899
                tunnel: [w2906 w2911] -> w2898
                tunnel: [w2905 w2910] -> w2897
                tunnel: [w2904 w2909] -> w2896
                tunnel: [w2903 w2908] -> w2895
                tunnel: w2894 -> [w2906 _]
                tunnel: w2893 -> [w2905 _]
                tunnel: w2892 -> [w2904 _]
                tunnel: w2891 -> [w2903 _]
                frame False {
                }
                frame True {
                  n1973 = Unbundle(w2916) -> (w2915:T31)
                  n1974 = call "isclickinwindow.vi"("Image Param"=w2915, "Point32"=w2914) -> ("4 Y"=w2908:i32, "3 Height"=w2909:i32, "2 X"=w2910:i32, "1 Width"=w2911:i32, "In image?"=w2913:bool)  [unwired: 1 in]
                  n1975 = Not(x=w2913) -> (.not. x?=w2912:bool)
                }
              }
            }
            n1976 = Not(x=w2866) -> (.not. x?=w2865:bool)
            n1977 = case shown="True" w2865 {
              tunnel: w2863 -> [_ w2930]
              tunnel: w2861 -> [_ w2929]
              tunnel: w2864 -> [_ w2928]
              tunnel: w2862 -> [_ w2927]
              frame False {
              }
              frame True {
                w2917 = FALSE ("Get Point")
                n1978 = local read "Scan lines (y)"() -> (w2932:u64)
                n1979 = disable-structure shown="Disabled" {
                  frame Disabled {
                  }
                  frame Enabled {
                  }
                }
                n1980 = local read "Actual MCL Inc (V)"() -> (w2926:dbl)
                n1981 = local read "Scan steps (MCL)"() -> (w2931:u64)
                n1982 = Divide "Y Pix/step"(x=w2927, y=w2932) -> (x/y=w2939:dbl)
                n1983 = Divide "Y V/pix"(x=w2926, y=w2939) -> (x/y=w2938:dbl)
                n1984 = Divide "Y half step offset"(x=w2926, y=2.0) -> (x/y=w2940:dbl)
                n1985 = Divide "X pix/step"(x=w2928, y=w2931) -> (x/y=w2937:dbl)